vi "HFRR ADV v038 new software.vi"() -> ()   [LabVIEW 2025] (continued)
                            n2653 = local write "START TEMP"(w3137) -> ()
                            n2654 = local write "Remarks :"(w3139) -> ()
                            n2655 = local write "Main Dashboard Buttons"(T1."Imaging" ("Main Dashboard Buttons")) -> ()
                            n2656 = local write "Main Tab"(T2."Adv Scar" ("Main Tab")) -> ()
                            n2657 = property on="FRICVALZ 2" class="Bool (strict)"("DisabledEnum"=w3138) -> ()  [unwired: 2 in, 2 out]
                            n2658 = property on="FRICVALZ 3" class="Bool (strict)"("DisabledEnum"=w3138) -> ()  [unwired: 2 in, 2 out]
                            n2659 = property on="FRICVALZ 4" class="Bool (strict)"("DisabledEnum"=w3138) -> ()  [unwired: 2 in, 2 out]
                          }
                          frame #1 {
                            n2660 = Wait (ms)(milliseconds to wait=u32 1500) -> ()  [unwired: 1 out]
                          }
                          frame #2 {
                            n2661 = local read "WriteHumidity"() -> (w3153:string[])
                            n2662 = Insert Into Array(array=w3153, new element="R;1" ("new element/subarray")) -> (w3151:string[])  [unwired: 1 in]
                            n2663 = local write "Due Write"("VC;0") -> ()
                            n2664 = local write "WriteHumidity"(w3151) -> ()
                          }
                          frame #3 {
                            n2665 = Wait (ms)(milliseconds to wait=u32 1500) -> ()  [unwired: 1 out]
                          }
                          frame #4 {
                            n2666 = local read "WriteHumidity"() -> (w3158:string[])
                            n2667 = Insert Into Array(array=w3158, new element="R;1" ("new element/subarray")) -> (w3157:string[])  [unwired: 1 in]
                            n2668 = local write "Due Write"("VC;0") -> ()
                            n2669 = local write "WriteHumidity"(w3157) -> ()
                          }
                          frame #5 {
                            n2670 = Wait (ms)(milliseconds to wait=u32 1500) -> ()  [unwired: 1 out]
                          }
                          frame #6 {
                            n2671 = local write "Due Write"("ST;0") -> ()
                          }
                          frame #7 {
                            n2672 = local write "measured_stroke"(0.0 ("measured_stroke")) -> ()
                            n2673 = Wait (ms)(milliseconds to wait=u32 1500) -> ()  [unwired: 1 out]
                          }
                          frame #8 {
                            n2674 = local write "Humidity"(FALSE ("Humidity")) -> ()
                            n2675 = local write "Due Write"("HE;0") -> ()
                          }
                        }
                      }
                    }
                    n2676 = Divide(x=w3122, y=w3121) -> (x/y=w3125:dbl)
                    n2677 = Multiply(x=w3125, y=100.0) -> (x*y=w3123:dbl)
                    n2678 = local write "Test Duration Status"(w3123) -> ()
                  }
                }
              }
              frame #2 {
                n2679 = case shown="True" "Heater Button" {
                  tunnel: [0.0 ("output") w3265] -> w3243
                  frame False {
                    w3246 = TRUE ("tmpchk")
                    n2680 = local read "TEMP"() -> (w3247:dbl)
                    n2681 = local write "Temp ini"(w3247) -> ()
                    n2682 = local write "Reset 4"(w3246) -> ()
                    n2683 = local write "tmpchk"(w3246) -> ()
                    n2684 = local write "reinit"(TRUE ("reinit")) -> ()
                    n2685 = local write "manual temp log"(TRUE ("manual temp log")) -> ()
                  }
                  frame True {
                    # "Logic to turn off\nthe heater when \ntemp is not rising.\nTime - 60 sec\nDelta t- 5°c"
                    n2686 = local read "Temp ini"() -> (w3254:dbl)
                    n2687 = local read "Auto Start Test"() -> (w3250:bool)
                    n2688 = Less?(x=w3254, y=53.0) -> (x < y?=w3252:bool)
                    n2689 = case shown="False" w3250 {
                      frame False {
                        n2690 = local read "Set Temp"() -> (w3274:dbl)
                        n2691 = local read "TEMP"() -> (w3273:dbl)
                        n2692 = Subtract(x=w3274, y=w3273) -> (x-y=w3272:dbl)
                        n2693 = Absolute Value(x=w3272) -> (abs(x)=w3271:dbl)
                        n2694 = Less?(x=w3271, y=0.5) -> (x < y?=w3269:bool)
                        n2695 = case shown="True" w3269 {
                          tunnel: "manual temp log" -> [_ w3275]
                          frame False {
                          }
                          frame True {
                            n2696 = case shown="True" w3275 {
                              selector: w3275 -> [_ w3276]
                              frame False {
                              }
                              frame True {
                                # "#Event log"
                                n2697 = Not(x=w3276) -> (.not. x?=w3277:bool)
                                n2698 = local write "manual temp log"(w3277) -> ()
                                n2699 = local read "EVENT LOG"() -> (w3280:string)
                                n2700 = call "Event Log.vi"("Content"="Target Temperature reached", "EVENT LOG"=w3280) -> ("EVENT LOG"=w3279:string)  [unwired: 8 in, 1 out]
                                n2701 = local write "EVENT LOG"(w3279) -> ()
                              }
                            }
                          }
                        }
                      }
                      frame True {
                        n2702 = local write "manual temp log"(TRUE ("manual temp log")) -> ()
                      }
                    }
                    n2703 = And(x="tmpchk", y=w3252) -> (x .and. y?=w3255:bool)
                    n2704 = case shown="True" w3255 {
                      frame False {
                      }
                      frame True {
                        n2705 = call "Elapsed Time8"("Time Target (s)"=300.0, "Reset"="Reset 4") -> ("Time has Elapsed"=w3282:bool)  [unwired: 10 in, 7 out]
                        n2706 = flat-sequence {
                          tunnel: w3282 -> [_]
                          frame #0 {
                            n2707 = local write "Reset 4"(FALSE ("Reset 4")) -> ()
                          }
                        }
                        n2708 = case shown="True" w3282 {
                          frame False {
                          }
                          frame True {
                            n2709 = local read "Temp ini"() -> (w3289:dbl)
                            n2710 = Add(x=w3289, y=5.0) -> (x+y=w3287:dbl)
                            n2711 = local read "TEMP"() -> (w3290:dbl)
                            n2712 = Greater?(x=w3290, y=w3287) -> (0:w3288:bool)
                            n2713 = case shown="False" w3288 {
                              frame False {
                                n2714 = local write "Heater Button"(FALSE ("Heater Button")) -> ()
                              }
                              frame True {
                                n2715 = local write "tmpchk"(FALSE ("tmpchk")) -> ()
                              }
                            }
                          }
                        }
                      }
                    }
                    n2716 = local read "Set Temp"() -> (w3263:dbl)
                    n2717 = local read "TEMP"() -> (w3257:dbl)
                    n2718 = call-poly <vilib>:"PID.vi"("reinitialize? (F)"="reinit", "dt (s)"=-1.0, "process variable"=w3257, "setpoint"=w3263) -> ("output"=w3260:dbl)  [unwired: 6 in, 1 out]
                    n2719 = Subtract(x=w3263, y=w3257) -> (x-y=w3264:dbl)
                    n2720 = Add(x=w3263, y=0.5) -> (x+y=w3261:dbl)
                    n2721 = Greater Or Equal?(x=w3257, y=w3261) -> ()  [unwired: 1 out]
                    n2722 = Select(t=0.0, s=FALSE, f=w3260) -> (s? t:f=w3259:dbl)
                    "PID output" <- w3259
                    n2723 = flat-sequence {
                      tunnel: w3259 -> [w3293]
                      tunnel: [w3293] -> w3265
                      frame #0 {
                        n2724 = local write "reinit"(FALSE ("reinit")) -> ()
                      }
                    }
                    n2725 = Bundle(w3264, "output"=w3259, "TEMP"=w3257) -> ()  [unwired: 1 in, 1 out]
                  }
                }
                "PID-out" <- w3243
              }
              frame #3 {
                n2726 = local read "TEMP"() -> (w3295:dbl)
                n2727 = Greater Or Equal?(x=w3295, y="Set Temp 2") -> (x >= y?=w3300:bool)
                n2728 = case shown="True" w3300 {
                  tunnel: [FALSE TRUE] -> w3298
                  frame False {
                  }
                  frame True {
                  }
                }
                "Status 13" <- w3298
                n2729 = And(x=w3298, y="trip1 8") -> (x .and. y?=w3297:bool)
                n2730 = case shown="True" w3297 {
                  frame False {
                    n2731 = local write "Heater Trip Temp"(TRUE ("Heater Trip Temp")) -> ()
                  }
                  frame True {
                    w3303 = FALSE ("OK Button 2")
                    n2732 = case shown="True" "Heater Trip Temp" {
                      selector: "Heater Trip Temp" -> [_ w3305]
                      frame False {
                      }
                      frame True {
                        n2733 = Not(x=w3305) -> (.not. x?=w3304:bool)
                        n2734 = local read "EVENT LOG"() -> (w3308:string)
                        n2735 = local write "Heater Trip Temp"(w3304) -> ()
                        n2736 = call "Event Log.vi"("Content"="Heater Trip", "EVENT LOG"=w3308) -> ("EVENT LOG"=w3307:string)  [unwired: 8 in, 1 out]
                        n2737 = local write "EVENT LOG"(w3307) -> ()
                      }
                    }
                    n2738 = local write "RUN"(w3303) -> ()
                    n2739 = property on="Auto Start Test" class="Bool (strict)"("Value"=w3303) -> ()  [unwired: 2 in, 2 out]
                    n2740 = local write "Heater Button"(w3303) -> ()
                  }
                }
              }
            }
            n2741 = case shown="False" w3010 {
              frame False {
                n2742 = disable-structure shown="Disabled" {
                  frame Disabled {
                    n2743 = stacked-sequence {
                      frame #0 {
                        n2744 = local write "RUN"(FALSE ("OK Button 2")) -> ()
                      }
                      frame #1 {
                      }
                    }
                  }
                  frame Enabled {
                  }
                }
              }
              frame True {
              }
            }
          }
        }
        n2745 = local read "Reset Graph"() -> (w2903:bool)
        n2746 = case shown="True" w2903 {
          selector: w2903 -> [_ w2920]
          frame False {
          }
          frame True {
            w2934 = 0.0 ("X Scale.Range:Maximum")
            n2747 = Not(x=w2920) -> (.not. x?=w2919:bool)
            n2748 = local write "Reset Graph"(w2919) -> ()
            n2749 = property on="Electrical Contact Resistance ( % )" class="WFChart (strict)"("XScale.Maximum"=600.0 ("X Scale.Range:Maximum"), "XScale.Minimum"=0.0 ("X Scale.Range:Minimum"), "YScale.Maximum"=100.0 ("Y Scale.Range:Maximum"), "YScale.Minimum"=0.0 ("Y Scale.Range:Minimum")) -> ()  [unwired: 2 in, 2 out]
            n2750 = property on="Frictional Force ( N )" class="WFChart (strict)"("XScale.Maximum"=600.0 ("X Scale.Range:Maximum"), "XScale.Minimum"=0.0 ("X Scale.Range:Minimum"), "YScale.Maximum"=100.0 ("Y Scale.Range:Maximum"), "YScale.Minimum"=0.0 ("Y Scale.Range:Minimum")) -> ()  [unwired: 2 in, 2 out]
            n2751 = property on="Temperature ( Deg C )" class="WFChart (strict)"("XScale.Maximum"=600.0 ("X Scale.Range:Maximum"), "XScale.Minimum"=0.0 ("X Scale.Range:Minimum"), "YScale.Maximum"=100.0 ("Y Scale.Range:Maximum"), "YScale.Minimum"=0.0 ("Y Scale.Range:Minimum")) -> ()  [unwired: 2 in, 2 out]
            n2752 = property on="Stroke ( mm )" class="WFChart (strict)"("XScale.Maximum"=600.0 ("X Scale.Range:Maximum"), "XScale.Minimum"=0.0 ("X Scale.Range:Minimum"), "YScale.Maximum"=100.0 ("Y Scale.Range:Maximum"), "YScale.Minimum"=0.0 ("Y Scale.Range:Minimum")) -> ()  [unwired: 2 in, 2 out]
            n2753 = property on="Coefficient of Friction" class="WFChart (strict)"("XScale.Maximum"=600.0 ("X Scale.Range:Maximum"), "XScale.Minimum"=0.0 ("X Scale.Range:Minimum"), "YScale.Maximum"=100.0 ("Y Scale.Range:Maximum"), "YScale.Minimum"=0.0 ("Y Scale.Range:Minimum")) -> ()  [unwired: 2 in, 2 out]
            n2754 = property on="Electrical Contact Resistance ( % )" class="WFChart (strict)"("XScale.Minimum"=0.0 ("X Scale.Range:Minimum"), "XScale.Maximum"=600.0 ("X Scale.Range:Maximum"), "YScale.Minimum"=0.0 ("Y Scale.Range:Minimum"), "YScale.Maximum"=100.0 ("Y Scale.Range:Maximum")) -> ()  [unwired: 2 in, 2 out]
            n2755 = property on="Temperature ( Deg C )" class="WFChart (strict)"("XScale.Minimum"=0.0 ("X Scale.Range:Minimum"), "XScale.Maximum"=600.0 ("X Scale.Range:Maximum"), "YScale.Minimum"=0.0 ("Y Scale.Range:Minimum"), "YScale.Maximum"=100.0 ("Y Scale.Range:Maximum")) -> ()  [unwired: 2 in, 2 out]
            n2756 = property on="Coefficient of Friction" class="WFChart (strict)"("XScale.Minimum"=0.0 ("X Scale.Range:Minimum"), "XScale.Maximum"=600.0 ("X Scale.Range:Maximum"), "YScale.Maximum"=1.0 ("X Scale.Range:Minimum"), "YScale.Minimum"=0.0 ("X Scale.Range:Minimum")) -> ()  [unwired: 2 in, 2 out]
            n2757 = property on="Frictional Force ( N )" class="WFChart (strict)"("XScale.Maximum"=600.0 ("X Scale.Range:Maximum"), "XScale.Minimum"=w2934, "YScale.Maximum"=10.0 ("Y Scale.Range:Maximum"), "YScale.Minimum"=w2934) -> ()  [unwired: 2 in, 2 out]
            n2758 = property on="Stroke ( mm )" class="WFChart (strict)"("XScale.Maximum"=600.0 ("X Scale.Range:Maximum"), "XScale.Minimum"=0.0 ("X Scale.Range:Minimum"), "YScale.Maximum"=100.0 ("Y Scale.Range:Maximum"), "YScale.Minimum"=0.0 ("Y Scale.Range:Minimum")) -> ()  [unwired: 2 in, 2 out]
            n2759 = property on="Humidity ( %RH ) 2" class="WFChart (strict)"("XScale.Maximum"=600.0 ("X Scale.Range:Maximum"), "XScale.Minimum"=0.0 ("X Scale.Range:Minimum"), "YScale.Maximum"=100.0 ("Y Scale.Range:Maximum"), "YScale.Minimum"=0.0 ("Y Scale.Range:Minimum")) -> ()  [unwired: 2 in, 2 out]
          }
        }
      }
      frame "Compare Files" {
        # "Elapsed time\ncof\nstroke\nAir temp\nTemp\nHumidity"
        n2760 = case shown="True" "RSTV1 2" {
          frame False {
          }
          frame True {
            n2761 = property on="Humidity ( %RH )" class="XYGraph (strict)"("Y Scale.Display Format:Precision"=u8 0 ("Y Scale.Format & Precision:Precision")) -> ()  [unwired: 2 in, 2 out]
            n2762 = property on="Humidity ( %RH )" class="XYGraph (strict)"("X Scale.Range:Minimum"=0.0, "X Scale.Range:Maximum"=75.0, "Y Scale.Range:Minimum"=48.0, "Y Scale.Range:Maximum"=58.0) -> ()  [unwired: 2 in, 2 out]
          }
        }
        n2763 = case shown="True" "RST CP 2" {
          frame False {
          }
          frame True {
            n2764 = property on="XY Graph 13" class="XYGraph (strict)"("Y Scale.Display Format:Precision"=u8 0 ("Y Scale.Format & Precision:Precision")) -> ()  [unwired: 2 in, 2 out]
            n2765 = property on="XY Graph 13" class="XYGraph (strict)"("X Scale.Range:Minimum"=0.0, "X Scale.Range:Maximum"=75.0, "Y Scale.Range:Minimum"=0.0, "Y Scale.Range:Maximum"=100.0) -> ()  [unwired: 2 in, 2 out]
          }
        }
        n2766 = case shown="True" "RST CP" {
          frame False {
          }
          frame True {
            n2767 = property on="Sample Temperature ( °C )" class="XYGraph (strict)"("Y Scale.Display Format:Precision"=u8 2 ("Y Scale.Format & Precision:Precision")) -> ()  [unwired: 2 in, 2 out]
            n2768 = property on="Sample Temperature ( °C )" class="XYGraph (strict)"("X Scale.Range:Minimum"=0.0, "X Scale.Range:Maximum"=75.0, "Y Scale.Range:Minimum"=58.0, "Y Scale.Range:Maximum"=62.0) -> ()  [unwired: 2 in, 2 out]
          }
        }
        n2769 = case shown="True" "RSTV1 3" {
          frame False {
          }
          frame True {
            n2770 = property on="Air Temperature  ( °C )" class="XYGraph (strict)"("Y Scale.Display Format:Precision"=u8 2 ("Y Scale.Format & Precision:Precision")) -> ()  [unwired: 2 in, 2 out]
            n2771 = property on="Air Temperature  ( °C )" class="XYGraph (strict)"("X Scale.Range:Minimum"=0.0 ("Y Scale.Range:Minimum"), "X Scale.Range:Maximum"=75.0 ("Y Scale.Range:Maximum"), "Y Scale.Range:Minimum"=20.0 ("X Scale.Range:Minimum"), "Y Scale.Range:Maximum"=26.0 ("X Scale.Range:Maximum")) -> ()  [unwired: 2 in, 2 out]
          }
        }
        n2772 = case shown="True" "RSTV1 4" {
          frame False {
          }
          frame True {
            n2773 = property on="Stroke ( mm )" class="XYGraph (strict)"("Y Scale.Display Format:Precision"=u8 2 ("Y Scale.Format & Precision:Precision")) -> ()  [unwired: 2 in, 2 out]
            n2774 = property on="Stroke ( mm )" class="XYGraph (strict)"("X Scale.Range:Minimum"=0.0 ("Y Scale.Range:Maximum"), "X Scale.Range:Maximum"=75.0 ("X Scale.Range:Minimum"), "Y Scale.Range:Minimum"=0.98, "Y Scale.Range:Maximum"=1.02) -> ()  [unwired: 2 in, 2 out]
          }
        }
        n2775 = case shown="True" "rstv2" {
          frame False {
          }
          frame True {
            n2776 = property on="Coefficient Of Friction" class="XYGraph (strict)"("Y Scale.Display Format:Precision"=u8 3 ("Y Scale.Format & Precision:Precision")) -> ()  [unwired: 2 in, 2 out]
            n2777 = property on="Coefficient Of Friction" class="XYGraph (strict)"("X Scale.Range:Minimum"=0.0 ("Y Scale.Range:Maximum"), "X Scale.Range:Maximum"=75.0, "Y Scale.Range:Minimum"=0.0, "Y Scale.Range:Maximum"=1.0 ("X Scale.Range:Minimum")) -> ()  [unwired: 2 in, 2 out]
          }
        }
        n2778 = case shown="True" "RST CP 3" {
          frame False {
          }
          frame True {
            n2779 = property on="Air Temp ( °C ) vs Humidity ( % RH )" class="XYGraph (strict)"("X Scale.Range:Minimum"=18.0, "X Scale.Range:Maximum"=28.0 ("X Scale.Range:Minimum"), "Y Scale.Range:Minimum"=30.0 ("X Scale.Range:Minimum"), "Y Scale.Range:Maximum"=70.0 ("X Scale.Range:Minimum")) -> ()  [unwired: 2 in, 2 out]
          }
        }
        n2780 = case shown="True" "OPEN 1" {
          frame False {
          }
          frame True {
            (unwired) 0  # existing file
            w3584 = "Choose a datalog file to open"  # prompt
            n2781 = local write "OPEN 1"(FALSE ("OPEN 1")) -> ()
            n2782 = String To Path(string="C:\\LAB-IQ\\Data\\") -> (path=w3569:path)
            n2783 = File Dialog(6:"*.dgf" ("pattern"), 7:w3584, 11:w3569) -> (0:w3567:errorcluster, 3:w3575:path)  [unwired: 4 in, 2 out]
            n2784 = Unbundle(w3567) -> ()  [unwired: 3 out]
            n2785 = Strip Path(path=w3575) -> (name=w3574:string)  [unwired: 1 out]
            n2786 = Path To String(path=w3575) -> (string=w3570:string)
            "string1" <- w3570
            n2787 = Match Pattern(string=w3574, regular expression=".dgf") -> (before substring=→"String Control":string)  [unwired: 1 in, 3 out]
            n2788 = Match Pattern(string=w3570, regular expression=".dgf" ("substring (\"\")")) -> (before substring=w3580:string)  [unwired: 1 in, 3 out]
            n2789 = Concatenate Strings(w3580, ".duf" ("Substring")) -> (w3576:string)
            n2790 = String To Path(string=w3576) -> (path=w3581:path)
            n2791 = call <vilib>:"Read Characters From File.vi"("file path (dialog if empty)"=w3581, "start of read offset (chars.:0)"=60 ("start of read offset (chars.: 0)")) -> ("character string"=→"String Control 2":string)  [unwired: 4 in, 3 out]
          }
        }
        n2792 = case shown="True" "OPEN 2" {
          frame False {
          }
          frame True {
            (unwired) 0  # existing file
            w3602 = "Choose a datalog file to open"  # prompt
            n2793 = local write "OPEN 2"(FALSE ("OPEN 1")) -> ()
            n2794 = String To Path(string="C:\\LAB-IQ\\Data\\") -> (path=w3587:path)
            n2795 = File Dialog(6:"*.dgf" ("pattern"), 7:w3602, 11:w3587) -> (0:w3585:errorcluster, 3:w3593:path)  [unwired: 4 in, 2 out]
            n2796 = Unbundle(w3585) -> ()  [unwired: 3 out]
            n2797 = Strip Path(path=w3593) -> (name=w3591:string)  [unwired: 1 out]
            n2798 = Path To String(path=w3593) -> (string=w3588:string)
            "string1 2" <- w3588
            n2799 = Match Pattern(string=w3591, regular expression=".dgf") -> (before substring=→"String Control 3":string)  [unwired: 1 in, 3 out]
            n2800 = Match Pattern(string=w3588, regular expression=".dgf" ("substring (\"\")")) -> (before substring=w3599:string)  [unwired: 1 in, 3 out]
            n2801 = Concatenate Strings(w3599, ".duf" ("Substring")) -> (w3596:string)
            n2802 = String To Path(string=w3596) -> (path=w3594:path)
            n2803 = call <vilib>:"Read Characters From File.vi"("file path (dialog if empty)"=w3594, "start of read offset (chars.:0)"=60 ("start of read offset (chars.: 0)")) -> ("character string"=→"String Control 4":string)  [unwired: 4 in, 3 out]
          }
        }
        n2804 = case shown="True" "OPEN 3" {
          frame False {
          }
          frame True {
            (unwired) 0  # existing file
            w3620 = "Choose a datalog file to open"  # prompt
            n2805 = local write "OPEN 3"(FALSE ("OPEN 1")) -> ()
            n2806 = String To Path(string="C:\\LAB-IQ\\Data\\") -> (path=w3605:path)
            n2807 = File Dialog(6:"*.dgf" ("pattern"), 7:w3620, 11:w3605) -> (0:w3603:errorcluster, 3:w3611:path)  [unwired: 4 in, 2 out]
            n2808 = Unbundle(w3603) -> ()  [unwired: 3 out]
            n2809 = Strip Path(path=w3611) -> (name=w3609:string)  [unwired: 1 out]
            n2810 = Path To String(path=w3611) -> (string=w3606:string)
            "string1 3" <- w3606
            n2811 = Match Pattern(string=w3609, regular expression=".dgf") -> (before substring=→"String Control 5":string)  [unwired: 1 in, 3 out]
            n2812 = Match Pattern(string=w3606, regular expression=".dgf" ("substring (\"\")")) -> (before substring=w3616:string)  [unwired: 1 in, 3 out]
            n2813 = Concatenate Strings(w3616, ".duf" ("Substring")) -> (w3613:string)
            n2814 = String To Path(string=w3613) -> (path=w3617:path)
            n2815 = call <vilib>:"Read Characters From File.vi"("file path (dialog if empty)"=w3617, "start of read offset (chars.:0)"=60 ("start of read offset (chars.: 0)")) -> ("character string"=→"String Control 6":string)  [unwired: 4 in, 3 out]
          }
        }
        n2816 = case shown="True" "OPEN 4" {
          frame False {
          }
          frame True {
            (unwired) 0  # existing file
            w3638 = "Choose a datalog file to open"  # prompt
            n2817 = local write "OPEN 4"(FALSE ("OPEN 1")) -> ()
            n2818 = String To Path(string="C:\\LAB-IQ\\Data\\") -> (path=w3623:path)
            n2819 = File Dialog(6:"*.dgf" ("pattern"), 7:w3638, 11:w3623) -> (0:w3621:errorcluster, 3:w3629:path)  [unwired: 4 in, 2 out]
            n2820 = Unbundle(w3621) -> ()  [unwired: 3 out]
            n2821 = Strip Path(path=w3629) -> (name=w3627:string)  [unwired: 1 out]
            n2822 = Path To String(path=w3629) -> (string=w3624:string)
            "string1 4" <- w3624
            n2823 = Match Pattern(string=w3627, regular expression=".dgf") -> (before substring=→"String Control 7":string)  [unwired: 1 in, 3 out]
            n2824 = Match Pattern(string=w3624, regular expression=".dgf" ("substring (\"\")")) -> (before substring=w3634:string)  [unwired: 1 in, 3 out]
            n2825 = Concatenate Strings(w3634, ".duf" ("Substring")) -> (w3631:string)
            n2826 = String To Path(string=w3631) -> (path=w3635:path)
            n2827 = call <vilib>:"Read Characters From File.vi"("file path (dialog if empty)"=w3635, "start of read offset (chars.:0)"=60 ("start of read offset (chars.: 0)")) -> ("character string"=→"String Control 8":string)  [unwired: 4 in, 3 out]
          }
        }
      }
      frame "About" {
        # "Elapsed time\ncof\nstroke\nmean pos\nTemp\nHumidity"
        n2828 = disable-structure shown="Disabled" {
          frame Disabled {
            n2829 = case shown="True" "Export" {
              frame False {
              }
              frame True {
                w3660 = "                                      " ("string")
                w3662 = "\r"
                (unwired) i16 6 ("width (-)")
                w3739 = "\r"
                w3671 = "\r"
                n2830 = local write "Export"(FALSE ("Export")) -> ()
                n2831 = local read "String 29"() -> (w3708:string)
                n2832 = local read "String 34"() -> (w3696:string)
                n2833 = local read "String 35"() -> (w3691:string)
                n2834 = local read "String 37"() -> (w3687:string)
                n2835 = local read "String 36"() -> (w3684:string)
                n2836 = local read "String 38"() -> (w3681:string)
                n2837 = local read "String 39"() -> (w3678:string)
                n2838 = Match Pattern(string=w3708, regular expression=".dwm") -> (before substring=w3704:string)  [unwired: 1 in, 3 out]
                "before substring" <- w3704
                n2839 = local read "S 38"() -> (w3699:string)
                n2840 = local read "S 39"() -> (w3692:string)
                n2841 = local read "Temperature before test 2"() -> (w3728:dbl)
                n2842 = local read "Temperature after test 2"() -> (w3733:dbl)
                n2843 = local read "Humidity before test 2"() -> (w3714:dbl)
                n2844 = local read "Humidity after test 2"() -> (w3729:dbl)
                n2845 = local read "MWSD 2"() -> (w3725:dbl)
                n2846 = local read "WS1.4 2"() -> (w3741:dbl)
                n2847 = local read "HCF 2"() -> (w3737:dbl)
                n2848 = local read "AVP 2"() -> (w3726:dbl)
                n2849 = Concatenate Strings("1," ("string"), w3699) -> (w3698:string)
                n2850 = Concatenate Strings("2," ("string"), w3696) -> (w3695:string)
                n2851 = Concatenate Strings("3," ("string"), w3692) -> (w3694:string)
                n2852 = Concatenate Strings("4," ("string"), w3691) -> (w3690:string)
                n2853 = Concatenate Strings("5," ("string"), w3687) -> (w3688:string)
                n2854 = Concatenate Strings("6," ("string"), w3684) -> (w3685:string)
                n2855 = Concatenate Strings("7," ("string"), w3681) -> (w3682:string)
                n2856 = Concatenate Strings("8," ("string"), w3678) -> (w3679:string)
                n2857 = local read "Sample ID"() -> (w3746:string)
                n2858 = case shown="\"xlx\"" "Select File Type" {
                  tunnel: w3704 -> [w3749 w3751 w3753]
                  tunnel: [w3747 w3752 w3754] -> w3703
                  frame "xlx" {
                    n2859 = Concatenate Strings(w3749, ".xls" ("string")) -> (w3747:string)
                  }
                  frame "csv" {
                    n2860 = Concatenate Strings(w3751, ".csv" ("string")) -> (w3752:string)
                  }
                  frame "txt" {
                    n2861 = Concatenate Strings(w3753, ".txt" ("string")) -> (w3754:string)
                  }
                }
                n2862 = local read "Test Date"() -> (w3745:string)
                n2863 = local read "String 45"() -> (w3659:string)
                n2864 = local read "String 31"() -> (w3744:string)
                n2865 = local read "String 32"() -> (w3743:string)
                n2866 = local read "TITTLE"() -> (w3667:string)
                n2867 = Number To Fractional String(number=w3714, width (-)=i16 6, precision (6)=i16 2) -> (F-format string=w3713:string)  [unwired: 1 in]
                n2868 = Number To Fractional String(number=w3728, width (-)=i16 6, precision (6)=i16 2) -> (F-format string=w3734:string)  [unwired: 1 in]
                n2869 = Number To Fractional String(number=w3729, width (-)=i16 6, precision (6)=i16 2) -> (F-format string=w3727:string)  [unwired: 1 in]
                n2870 = Number To Fractional String(number=w3733, width (-)=i16 6, precision (6)=i16 2) -> (F-format string=w3732:string)  [unwired: 1 in]
                n2871 = Number To Fractional String(number=w3725, width (-)=i16 6, precision (6)=i16 2) -> (F-format string=w3723:string)  [unwired: 1 in]
                n2872 = Number To Fractional String(number=w3726, width (-)=i16 6, precision (6)=i16 2) -> (F-format string=w3724:string)  [unwired: 1 in]
                n2873 = Number To Fractional String(number=w3737, width (-)=i16 6, precision (6)=i16 2) -> (F-format string=w3738:string)  [unwired: 1 in]
                n2874 = Number To Fractional String(number=w3741, precision (6)=i16 2) -> (F-format string=w3742:string)  [unwired: 2 in]
                n2875 = local read "s.NO"() -> (w3661:string)
                n2876 = Concatenate Strings("=" ("string"), w3667) -> (w3666:string)
                n2877 = Concatenate Strings("S.No," ("string"), "                                       Parameters" ("string")) -> (w3672:string)
                n2878 = Concatenate Strings(w3739, w3698, w3713, w3739, w3695, w3734, w3739, w3694, w3727, w3739, w3690, w3732, w3739, w3688, w3723, w3739, w3685, w3724, w3739, w3682, w3738, w3739, w3679, w3742) -> (w3701:string)
                n2879 = Concatenate Strings(w3671, "," ("string"), w3659, w3661, w3660, w3743, w3746, w3660, w3744, w3745, w3671) -> (w3669:string)
                n2880 = local read "Tested by"() -> (w3675:string)
                n2881 = local read "String 33"() -> (w3676:string)
                n2882 = Concatenate Strings("," ("string"), "                                                                             " ("string")) -> (w3664:string)
                n2883 = Concatenate Strings(w3666, w3662, w3669, w3662, w3672, w3701, w3662, w3664, w3676, w3675) -> (→"export":string)
                n2884 = String To Path(string=w3703) -> (path=w3710:path)
                n2885 = local read "export"() -> (w3705:string)
                n2886 = call <vilib>:"Write Characters To File.vi"("append to file? (new file:F)"=FALSE, "character string"=w3705, "file path (dialog if empty)"=w3710) -> ()  [unwired: 2 in, 1 out]
              }
            }
          }
          frame Enabled {
          }
        }
        n2887 = case shown="True" "OK Button 17" {
          frame False {
          }
          frame True {
            (unwired) 0  # existing file
            w3963 = "Choose a datalog file to open"  # prompt
            n2888 = local write "OK Button 17"(FALSE ("OK Button 17")) -> ()
            n2889 = local read "String"() -> (w3958:string)
            n2890 = String To Path(string=w3958) -> (path=w3959:path)
            n2891 = File Dialog(6:"*.duf" ("pattern"), 7:w3963, 11:w3959) -> (0:w3950:errorcluster, 3:w3969:path)  [unwired: 4 in, 2 out]
            n2892 = Unbundle(w3950) -> ()  [unwired: 3 out]
            n2893 = Open/Create/Replace File "Open File"(file path (use dialog)=w3969) -> (refnum out=w3961:refnum<file>)  [unwired: 5 in, 2 out]
            n2894 = Strip Path(path=w3969) -> (name=w3967:string)  [unwired: 1 out]
            n2895 = Path To String(path=w3969) -> (string=w3952:string)
            n2896 = while {
              tunnel: w3961 -> [w3973]
              i -> [w3970]
              stop <- w3971 continue-if-true
              (unwired) TRUE ("line mode (F)")
              n2897 = Read from Text File "Read File"(file (use dialog)=w3973) -> (text=w3972:string)  [unwired: 3 in, 3 out]
              n2898 = local write "Numeric 16"(w3970) -> ()
              n2899 = String Length(string=w3972) -> (length=w3975:i32)
              n2900 = Greater?(x=w3975, y=1) -> (0:w3971:bool)
            }
            n2901 = local write "String 29"(w3952) -> ()
            n2902 = Search and Replace String(input string=w3952, search string=".duf", replace string=".dgf" ("replace string (\"\")")) -> (result string=→"String Indicator 4":string)  [unwired: 5 in, 3 out]
            n2903 = Match Pattern(string=w3967, regular expression=".dwm") -> (before substring=w3951:string)  [unwired: 1 in, 3 out]
            "String Indicator" <- w3951
            n2904 = Match Pattern(string=w3952, regular expression=".dwm" ("substring (\"\")")) -> (before substring=w3953:string)  [unwired: 1 in, 3 out]
            "String Indicator 3" <- w3953
            n2905 = local write "TITTLE 2"(w3951) -> ()
            n2906 = String To Path(string=w3953) -> (path=w3960:path)
            "path" <- w3960
            n2907 = call <vilib>:"Read Characters From File.vi"("file path (dialog if empty)"=w3960, "start of read offset (chars.:0)"=60 ("start of read offset (chars.: 0)")) -> ("character string"=→"String Indicator 2":string)  [unwired: 4 in, 3 out]
          }
        }
        n2908 = call <vilib>:"Query Available Printers.vi"() -> ("system configured printers"=w3652:string[])  [unwired: 9 in, 2 out]
        "System Configured Printers 2" <- w3652
        n2909 = local read "OK Button 16"() -> (w3649:bool)
        n2910 = case shown="True" "OK Button 16" {
          frame False {
          }
          frame True {
            n2911 = stacked-sequence {
              frame #0 {
                n2912 = local read "Numeric 16"() -> (w3977:i32)
                n2913 = local write "Numeric 10"(w3977) -> ()
              }
              frame #1 {
                n2914 = local read "String 29"() -> (w3980:string)
                n2915 = String To Path(string=w3980) -> (path=w3979:path)
                n2916 = Open/Create/Replace File "Open File"(file path (use dialog)=w3979) -> (refnum out=w3981:refnum<file>)  [unwired: 5 in, 2 out]
                n2917 = for {
                  N: 16 -> [_]
                  tunnel: w3981 -> [w3988]
                  i -> [w3984]
                  (unwired) TRUE ("line mode (F)")
                  n2918 = Read from Text File "Read File"(file (use dialog)=w3988) -> (text=w3982:string)  [unwired: 3 in, 3 out]
                  n2919 = Match Pattern(string=w3982, regular expression="(") -> (after substring=w3987:string)  [unwired: 1 in, 3 out]
                  n2920 = Match Pattern(string=w3987, regular expression=")") -> (before substring=w3983:string)  [unwired: 1 in, 3 out]
                  n2921 = case shown="1" w3984 {
                    tunnel: w3983 -> [w3989 w3990 _ _ w3991 w3992 w3993 w3995 w3997 w3999 w4001 w4003 w4005 w4007 _]
                    tunnel: w3982 -> [_ _ _ _ _ _ _ _ _ _ _ _ _ _ _]
                    frame 0 {
                      "TITTLE" <- w3989
                    }
                    frame 1 {
                      "Sample ID" <- w3990
                    }
                    frame 2 {
                    }
                    frame 3 {
                    }
                    frame 4 {
                      "Test Date" <- w3991
                    }
                    frame 5 {
                      "Tested by" <- w3992
                    }
                    frame 6 {
                      n2922 = Fract/Exp String To Number(string=w3993) -> (number=→"Humidity before test 2":dbl)  [unwired: 3 in, 1 out]
                    }
                    frame 7 {
                      n2923 = Fract/Exp String To Number(string=w3995) -> (number=→"Temperature before test 2":dbl)  [unwired: 3 in, 1 out]
                    }
                    frame 8 {
                      n2924 = Fract/Exp String To Number(string=w3997) -> (number=→"Humidity after test 2":dbl)  [unwired: 3 in, 1 out]
                    }
                    frame 9 {
                      n2925 = Fract/Exp String To Number(string=w3999) -> (number=→"Temperature after test 2":dbl)  [unwired: 3 in, 1 out]
                    }
                    frame 10 {
                      n2926 = Fract/Exp String To Number(string=w4001) -> (number=→"MWSD 2":dbl)  [unwired: 3 in, 1 out]
                    }
                    frame 11 {
                      n2927 = Fract/Exp String To Number(string=w4003) -> (number=→"AVP 2":dbl)  [unwired: 3 in, 1 out]
                    }
                    frame 12 {
                      n2928 = Fract/Exp String To Number(string=w4005) -> (number=→"HCF 2":dbl)  [unwired: 3 in, 1 out]
                    }
                    frame 13 {
                      n2929 = Fract/Exp String To Number(string=w4007) -> (number=→"WS1.4 2":dbl)  [unwired: 3 in, 1 out]
                    }
                    frame 14, Default {
                    }
                  }
                }
              }
              frame #2 {
              }
            }
            n2930 = local write "OK Button 16"(FALSE ("OK Button 13")) -> ()
          }
        }
        n2931 = Index Array(array=w3652, index="Select Printer 3") -> (element=w3654:string)
        "Selected Printer" <- w3654
        n2932 = case shown="True" w3649 {
          frame False {
          }
          frame True {
            n2933 = flat-sequence {
              frame #0 {
              }
              frame #1 {
                n2934 = Wait (ms)(milliseconds to wait=u32 100) -> ()  [unwired: 1 out]
              }
              frame #2 {
                n2935 = local write "OK Button 16"(FALSE ("Print 3")) -> ()
              }
            }
          }
        }
        n2936 = case shown="True" "Print" {
          tunnel: w3654 -> [_ w3946]
          frame False {
          }
          frame True {
            (unwired) i16 6 ("width (-)")
            (unwired) "TESTED BY : "
            (unwired) "TESTED DATE :"
            (unwired) "SAMPLE ID : "
            (unwired) "SAMPLE DESIGN : "
            w3904 = "\r"
            w3921 = "\r"
            # "add image"
            n2937 = local read "Sample ID"() -> (w3894:string)
            n2938 = local read "Tested by"() -> (w3897:string)
            n2939 = local read "String 34"() -> (w3884:string)
            n2940 = local read "String 45"() -> (w3864:string)
            n2941 = local read "String 35"() -> (w3879:string)
            n2942 = local read "String 37"() -> (w3877:string)
            n2943 = local read "String 32"() -> (w3899:string)
            n2944 = local read "String 36"() -> (w3874:string)
            n2945 = local read "String 31"() -> (w3898:string)
            n2946 = local read "Test Date"() -> (w3895:string)
            n2947 = local read "String 33"() -> (w3900:string)
            n2948 = local read "String 38"() -> (w3870:string)
            n2949 = local read "String 39"() -> (w3867:string)
            n2950 = local write "Print"(FALSE ("Print FF")) -> ()
            n2951 = local read "S 39"() -> (w3882:string)
            n2952 = local read "S 38"() -> (w3889:string)
            n2953 = local read "Temperature before test 2"() -> (w3920:dbl)
            n2954 = local read "Temperature after test 2"() -> (w3910:dbl)
            n2955 = local read "Humidity before test 2"() -> (w3935:dbl)
            n2956 = local read "Humidity after test 2"() -> (w3919:dbl)
            n2957 = local read "MWSD 2"() -> (w3924:dbl)
            n2958 = local read "WS1.4 2"() -> (w3902:dbl)
            n2959 = Concatenate Strings("2)" ("string"), w3884) -> (w3885:string)
            n2960 = Concatenate Strings("3)" ("string"), w3882) -> (w3883:string)
            n2961 = Concatenate Strings("1)" ("string"), w3889) -> (w3888:string)
            n2962 = Concatenate Strings("4)" ("string"), w3879) -> (w3880:string)
            n2963 = Concatenate Strings("5)" ("string"), w3877) -> (w3876:string)
            n2964 = Concatenate Strings("6)" ("string"), w3874) -> (w3873:string)
            n2965 = Concatenate Strings("7)" ("string"), w3870) -> (w3871:string)
            n2966 = Concatenate Strings("8)" ("string"), w3867) -> (w3868:string)
            n2967 = local read "HCF 2"() -> (w3906:dbl)
            n2968 = local read "AVP 2"() -> (w3923:dbl)
            n2969 = local read "s.NO"() -> (w3865:string)
            n2970 = call <vilib>:"New Report.vi"("report type"=enum16{"Standard Report", "HTML"}."Standard Report") -> ("report out"=w3944:refnum<class "NI_report.lvclass">, "error out"=w3943:errorcluster)  [unwired: 13 in]
            n2971 = local read "TITTLE"() -> (w3896:string)
            n2972 = Concatenate Strings(w3921, w3864, w3865, w3921, w3899, w3894, w3921, w3898, w3895, w3921, w3900, w3897, w3921) -> (w3914:string)
            "test by" <- w3914
            n2973 = Number To Fractional String(number=w3920, width (-)=i16 6, precision (6)=i16 2) -> (F-format string=w3909:string)  [unwired: 1 in]
            n2974 = Number To Fractional String(number=w3919, width (-)=i16 6, precision (6)=i16 2) -> (F-format string=w3922:string)  [unwired: 1 in]
            n2975 = Number To Fractional String(number=w3935, width (-)=i16 6, precision (6)=i16 2) -> (F-format string=w3940:string)  [unwired: 1 in]
            n2976 = Number To Fractional String(number=w3924, width (-)=i16 6, precision (6)=i16 2) -> (F-format string=w3926:string)  [unwired: 1 in]
            n2977 = Number To Fractional String(number=w3910, width (-)=i16 6, precision (6)=i16 2) -> (F-format string=w3911:string)  [unwired: 1 in]
            n2978 = Number To Fractional String(number=w3923, width (-)=i16 6, precision (6)=i16 2) -> (F-format string=w3925:string)  [unwired: 1 in]
            n2979 = Number To Fractional String(number=w3906, width (-)=i16 6, precision (6)=i16 2) -> (F-format string=w3905:string)  [unwired: 1 in]
            n2980 = Number To Fractional String(number=w3902, precision (6)=i16 2) -> (F-format string=w3901:string)  [unwired: 2 in]
            n2981 = call-dynamic "Set Report Header Text.vi"("report in"=w3944, "center header text"=w3896, "error in (no error)"=w3943) -> ("report out"=w3915:refnum<class "NI_report.lvclass">, "error out"=w3916:errorcluster)  [unwired: 11 in]
            n2982 = Concatenate Strings(w3904, w3888, w3940, w3904, w3885, w3909, w3904, w3883, w3922, w3904, w3880, w3911, w3904, w3876, w3926, w3904, w3873, w3925, w3904, w3871, w3905, w3904, w3868, w3901) -> (w3892:string)
            "export 2" <- w3892
            n2983 = call-poly <vilib>:"Append Report Text.vi"("report in"=w3915, "text"=w3914, "error in (no error)"=w3916) -> ("report out"=w3918:refnum<class "NI_report.lvclass">, "error out"=w3917:errorcluster)  [unwired: 9 in, 2 out]
            n2984 = local read "test by"() -> (w3891:string)
            n2985 = local read "TITTLE"() -> (w3893:string)
            n2986 = call-poly <vilib>:"Append Report Text.vi"("report in"=w3918, "error in (no error)"=w3917) -> ("report out"=w3939:refnum<class "NI_report.lvclass">, "error out"=w3937:errorcluster)  [unwired: 10 in, 2 out]
            n2987 = Concatenate Strings(w3893, w3892, w3891) -> (→"output":string)
            n2988 = call-poly <vilib>:"Append Report Text.vi"("report in"=w3939, "text"=w3892, "error in (no error)"=w3937) -> ("report out"=w3938:refnum<class "NI_report.lvclass">, "error out"=w3936:errorcluster)  [unwired: 9 in, 2 out]
            n2989 = call-dynamic "Print Report.vi"("report in"=w3938, "printer name (default)"=w3946, "error in (no error)"=w3936) -> ("report out"=w3948:refnum<class "NI_report.lvclass">, "error out"=w3949:errorcluster)  [unwired: 11 in]
            n2990 = call-dynamic "Dispose Report.vi"("report in"=w3948, "error in (no error)"=w3949) -> ()  [unwired: 13 in, 1 out]
          }
        }
        n2991 = case shown="True" "Print 2" {
          frame False {
          }
          frame True {
            n2992 = flat-sequence {
              frame #0 {
                n2993 = local read "s.NO"() -> (→"s.NO 2":string)
                n2994 = Wait (ms)(milliseconds to wait=u32 20) -> ()  [unwired: 1 out]
                n2995 = local read "Sample ID  3"() -> (→"Sample ID  6":string)
                n2996 = local read "Sample ID  4"() -> (→"Sample ID  7":string)
                n2997 = local read "Sample ID"() -> (→"Sample ID  2":string)
                n2998 = local read "Tested by"() -> (→"Tested by 2":string)
                n2999 = local read "Test Date"() -> (→"Test Date 2":string)
                n3000 = local read "Humidity after test 3"() -> (→"Humidity after test 4":dbl)
                n3001 = local read "Ref A Test Date :"() -> (→"TITTLE 4":string)
                n3002 = local read "Temperature before test 3"() -> (w3771:dbl)
                n3003 = local read "Temperature before test 3"() -> (→"Temperature after test 5":dbl)
                n3004 = local read "Temperature after test 3"() -> (→"Temperature after test 4":dbl)
                n3005 = local read "Humidity before test 3"() -> (→"Humidity before test 4":dbl)
                n3006 = local write "Temperature before test 3"(w3771) -> ()
                n3007 = local read "image data"() -> (w3762:T16)
                n3008 = String To Path(string="C:\\LAB-IQ\\im\\Temp_resized.jpg") -> (path=w3763:path)
                "path 2" <- w3763
                n3009 = call <vilib>:"Write JPEG File.vi"("image data"=w3762, "path to JPEG file"=w3763) -> ()  [unwired: 8 in, 2 out]
                "Ref A Test Date :" <- "Ref A Test Date :"
                "Ref B Test Date :" <- "Ref B Test Date :"
                "Ref B Scar Value :" <- "Ref B Scar Value :"
                "Ref A Scar Value :" <- "Ref A Scar Value :"
              }
              frame #1 {
                (unwired) HTML_Report_Image_Alignment."MIDDLE" ("alignment (default)")
                w3799 = u16 0 items=["portrait", "landscape"] ("orientation (portrait)")
                (unwired) HTML_Report_Image_Alignment."ABSMIDDLE" ("alignment (default)")
                (unwired) "TESTED BY : "
                (unwired) "TESTED DATE :"
                (unwired) "SAMPLE ID : "
                (unwired) "SAMPLE DESIGN : "
                w3832 = "\r"
                # "add image"
                n3010 = Wait (ms)(milliseconds to wait=u32 20) -> ()  [unwired: 1 out]
                n3011 = local read "Sample ID  2"() -> (w3825:string)
                n3012 = local read "Wear Scar X"() -> (w3797:dbl)
                "Length ( microns ) 2" <- w3797
                n3013 = local read "Wear Scar Y"() -> (w3796:dbl)
                "Wear Scar Y ( microns ) :" <- w3796
                n3014 = local read "Test Date 2"() -> (w3826:string)
                n3015 = local read "Tested by 2"() -> (w3827:string)
                n3016 = local read "String 46"() -> (w3823:string)
                n3017 = local read "String 48"() -> (w3829:string)
                n3018 = local read "String 47"() -> (w3828:string)
                n3019 = local read "String 49"() -> (w3830:string)
                n3020 = local read "String 10"() -> (w3783:string)
                n3021 = local read "s.NO 2"() -> (w3824:string)
                n3022 = Add(x=w3797, y=w3796) -> (x+y=w3795:dbl)
                n3023 = call <vilib>:"New Report.vi"("report type"=enum16{"Standard Report", "HTML"}."HTML") -> ("report out"=w3803:refnum<class "NI_report.lvclass">, "error out"=w3801:errorcluster)  [unwired: 13 in]
                n3024 = Concatenate Strings(w3832, w3823, w3824, w3832, w3829, w3825, w3832, w3828, w3826, w3832, w3830, w3827, w3832) -> (→"test by 2":string)
                n3025 = Concatenate Strings("C:\\LAB-IQ\\Data\\" ("string"), w3783, ".jpg" ("string")) -> ()  [unwired: 1 out]
                n3026 = Divide(x=w3795, y=2.0) -> (x/y=→"Mean Wear ( microns) :":dbl)
                n3027 = call-dynamic "Set Report Orientation.vi"("report in"=w3803, "orientation (portrait)"=w3799, "error in (no error)"=w3801) -> ("report out"=w3802:refnum<class "NI_report.lvclass">, "error out"=w3800:errorcluster)  [unwired: 11 in]
                n3028 = for {
                  N: 5 -> [_]
                  tunnel: w3802 -> [w3853]
                  tunnel: [w3852] -> w3781
                  tunnel: w3800 -> [w3851]
                  tunnel: [w3850] -> w3780
                  n3029 = call-dynamic "Set Report Tab Width.vi"("report in"=w3853, "error in (no error)"=w3851) -> ("report out"=w3852:refnum<class "NI_report.lvclass">, "error out"=w3850:errorcluster)  [unwired: 12 in]
                }
                n3030 = local read "TITTLE"() -> (w3798:string)
                n3031 = call-dynamic "Set Report Header Text.vi"("report in"=w3781, "center header text"=w3798, "error in (no error)"=w3780) -> ("report out"=w3819:refnum<class "NI_report.lvclass">, "error out"=w3818:errorcluster)  [unwired: 11 in]
                n3032 = for {
                  N: 1 -> [_]
                  tunnel: [w3857] -> w3805
                  tunnel: [w3856] -> w3804
                  tunnel: w3819 -> [w3855]
                  tunnel: w3818 -> [w3854]
                  n3033 = call-dynamic "New Report Line.vi"("report in"=w3855, "error in (no error)"=w3854) -> ("report out"=w3857:refnum<class "NI_report.lvclass">, "error out"=w3856:errorcluster)  [unwired: 12 in]
                }
                n3034 = for {
                  N: 2 -> [_]
                  tunnel: [w3849] -> w3811
                  tunnel: [w3848] -> w3810
                  tunnel: w3805 -> [w3847]
                  tunnel: w3804 -> [w3846]
                  n3035 = call-dynamic "New Report Line.vi"("report in"=w3847, "error in (no error)"=w3846) -> ("report out"=w3849:refnum<class "NI_report.lvclass">, "error out"=w3848:errorcluster)  [unwired: 12 in]
                }
                n3036 = for {
                  N: 25 -> [_]
                  tunnel: w3811 -> [w3845]
                  tunnel: w3810 -> [w3843]
                  tunnel: [w3844] -> w3814
                  tunnel: [w3842] -> w3813
                  n3037 = call-dynamic "Set Report Tab Width.vi"("report in"=w3845, "error in (no error)"=w3843) -> ("report out"=w3844:refnum<class "NI_report.lvclass">, "error out"=w3842:errorcluster)  [unwired: 12 in]
                }
                n3038 = control-ref of="Tab Control 9"() -> (w3809:refnum<vi>)
                n3039 = call-dynamic "Append Control Image to Report.vi"("report in"=w3814, "alignment (default)"=HTML_Report_Image_Alignment."ABSMIDDLE", "ctrl reference"=w3809, "error in (no error)"=w3813) -> ("report out"=w3808:refnum<class "NI_report.lvclass">, "error out"=w3807:errorcluster)  [unwired: 8 in, 2 out]
                n3040 = for {
                  N: 3 -> [_]
                  tunnel: [w3841] -> w3792
                  tunnel: [w3840] -> w3791
                  tunnel: w3808 -> [w3839]
                  tunnel: w3807 -> [w3838]
                  n3041 = call-dynamic "New Report Line.vi"("report in"=w3839, "error in (no error)"=w3838) -> ("report out"=w3841:refnum<class "NI_report.lvclass">, "error out"=w3840:errorcluster)  [unwired: 12 in]
                }
                n3042 = for {
                  N: 100 -> [_]
                  tunnel: w3792 -> [w3837]
                  tunnel: w3791 -> [w3835]
                  tunnel: [w3836] -> w3788
                  tunnel: [w3834] -> w3786
                  n3043 = call-dynamic "Set Report Tab Width.vi"("report in"=w3837, "error in (no error)"=w3835) -> ("report out"=w3836:refnum<class "NI_report.lvclass">, "error out"=w3834:errorcluster)  [unwired: 12 in]
                }
                n3044 = String To Path(string="C:\\LAB-IQ\\im\\Temp_resized.jpg") -> (path=w3778:path)
                n3045 = call-poly <vilib>:"Append Image to Report.vi"("report in"=w3788, "path or URL of image"=w3778, "error in (no error)"=w3786) -> ("report out"=w3787:refnum<class "NI_report.lvclass">, "error out"=w3785:errorcluster)  [unwired: 9 in, 2 out]
                n3046 = call-poly <vilib>:"Open HTML Report in Browser.vi"("report in"=w3787, "error in (no error)"=w3785) -> ("report out"=w3822:refnum<class "NI_report.lvclass">, "error out"=w3821:errorcluster)  [unwired: 11 in, 1 out]
                n3047 = call-dynamic "Dispose Report.vi"("report in"=w3822, "error in (no error)"=w3821) -> ()  [unwired: 13 in, 1 out]
              }
              frame #2 {
              }
              frame #3 {
                n3048 = disable-structure shown="Disabled" {
                  frame Disabled {
                    n3049 = local read "String 10"() -> (w3862:string)
                    n3050 = Concatenate Strings("C:\\LAB-IQ-NXT\\Data\\" ("string"), w3862, ".jpg" ("string")) -> (w3860:string)
                    n3051 = String To Path(string=w3860) -> (path=w3859:path)
                    n3052 = Delete(path (use dialog)=w3859) -> ()  [unwired: 4 in, 3 out]
                  }
                  frame Enabled {
                  }
                }
                n3053 = local write "Print 2"(FALSE ("Print")) -> ()
              }
            }
          }
        }
      }
    }
    n3054 = Wait (ms)(milliseconds to wait=u32 50) -> ()  [unwired: 1 out]
    n3055 = Wait (ms)(milliseconds to wait=u32 50) -> ()  [unwired: 1 out]
    n3056 = local read "Quit"() -> (w2196:bool)
  }
  n3057 = VISA Close(VISA resource name=w41, error in (no error)=w40) -> ()  [unwired: 1 out]
  n3058 = while {
    stop <- w4013 stop-if-true
    n3059 = local read "Auto Start Test"() -> (w4011:bool)
    n3060 = local read "RUN"() -> (w4010:bool)
    n3061 = Wait (ms)(milliseconds to wait=u32 1000) -> ()  [unwired: 1 out]
    n3062 = Or(x=w4010, y=w4011) -> (x .or. y?=w4009:bool)
    n3063 = case shown="True" w4009 {
      frame False {
      }
      frame True {
        n3064 = local read "LVDT STROKE Actual"() -> (w4014:dbl)
        n3065 = In Range and Coerce(upper limit=1.2, x=w4014, lower limit=0.6) -> (In Range?=w4017:bool)  [unwired: 1 out]
        n3066 = call-poly <vilib>:"Random Number (Range).vi"("lower bound (0)"=0.998 ("upper bound (100)"), "upper bound (100)"=1.003) -> ("number"=w4015:dbl)  [unwired: 9 in]
        n3067 = case shown="True" w4017 {
          tunnel: [w4022 w4023] -> w4016
          tunnel: w4015 -> [_ w4023]
          tunnel: w4014 -> [w4022 _]
          frame False {
          }
          frame True {
          }
        }
        "LVDT STROKE DISPLAY" <- w4016
      }
    }
    n3068 = local read "Quit"() -> (w4013:bool)
  }
  n3069 = while {
    tunnel: [w4040] -> w49
    shift-right: [w4033] -> _
    shift-left: 0.0 -> [w4036]
    shift-right: [w4032] -> _
    shift-left: 0.0 -> [w4035]
    shift-right: [w4031] -> _
    shift-left: 100.0 ("vc_cmd") -> [w4034]
    stop <- w4040 stop-if-true
    # "PID LOGIC"
    n3070 = local read "run test Calibration"() -> (w4028:bool)
    n3071 = local read "RUN"() -> (w4038:bool)
    n3072 = local read "Auto Start Temp"() -> (w4029:bool)
    n3073 = local read "Auto Start Test"() -> (w4037:bool)
    n3074 = local read "START TEMP"() -> (w4027:bool)
    n3075 = And(x=w4029, y=w4037) -> (x .and. y?=w4030:bool)
    n3076 = Or(x=w4038, y=w4030) -> (x .or. y?=w4039:bool)
    n3077 = And(x=w4039, y=w4027) -> (x .and. y?=w4026:bool)
    n3078 = And(x=w4028, y=w4027) -> (x .and. y?=w4025:bool)
    n3079 = Or(x=w4025, y=w4026) -> (x .or. y?=w4024:bool)
    n3080 = Wait (ms)(milliseconds to wait="milliseconds to wait") -> ()  [unwired: 1 out]
    n3081 = case shown="True" w4024 {
      tunnel: [400.0 ("out_vc_cmd") w4059] -> w4031
      tunnel: [w4043 w4061] -> w4032
      tunnel: [w4043 w4060] -> w4033
      tunnel: w4036 -> [_ w4050]
      tunnel: w4035 -> [_ w4049]
      tunnel: w4034 -> [_ w4048]
      tunnel: w4028 -> [_ w4044]
      frame False {
        w4043 = 0.0 ("error_out")
      }
      frame True {
        n3082 = case shown="True" w4044 {
          tunnel: [w4068 1.0] -> w4046
          frame False {
            n3083 = local read "Set Strk"() -> (w4067:dbl)
            n3084 = Add(x=w4067, y="Add up Stroke") -> (x+y=w4068:dbl)
          }
          frame True {
          }
        }
        n3085 = local read "LVDT STROKE"() -> (w4045:dbl)
        n3086 = formula code="// Zero-Hardcode Explicit Positional-Form PID Engine\n// Inputs: target_stroke, measured_stroke, dt, prev_error, integral_accumulator_in, prev_vc_cmd\n//         kp, ki, kd, max_step_change, max_amplitude, min_amplitude, startup_cmd\n// Outputs: vc_cmd, error_out, out_error, integral_accumulator_out, out_vc_cmd\n\n// 1. Calculate Tracking Error\nfloat current_error = target_stroke - measured_stroke;\nerror_out = current_error;\n\n// 2. Compute Proportional Term\nfloat p_term = kp * current_error;\n\n// 3. Compute Derivative Term\nfloat d_term = 0.0;\nif (dt > 0.0) {\n    d_term = kd * ((current_error - prev_error) / dt);\n}\n\n// 4. Update and Accumulate Integral Term\nfloat current_integral = integral_accumulator_in + (current_error * dt);\nfloat i_term = ki * current_integral;\n\n// 5. Calculate Ideal Target Command (Anchored by startup baseline)\nfloat ideal_command = startup_cmd + p_term + i_term + d_term;\n\n// 6. Apply Loop Rate Limiting FIRST \n// (Forces the command to climb gradually from prev_vc_cmd instead of jumping straight to max)\nfloat raw_adjustment = ideal_command - prev_vc_cmd;\n\nif (raw_adjustment > max_step_change) {\n    raw_adjustment = max_step_change;\n} else if (raw_adjustment < -max_step_change) {\n    raw_adjustment = -max_step_change;\n}\n\nfloat next_vc_cmd = prev_vc_cmd + raw_adjustment;\n\n// 7. Anti-Windup Protection & Final Output Safety Safeguard Clamping\n// (Back-calculating based on what we are ACTUALLY outputting)\nif (next_vc_cmd > max_amplitude) {\n    float excess = next_vc_cmd - max_amplitude;\n    if (ki > 0.0) {\n        current_integral -= excess / ki;\n    }\n    next_vc_cmd = max_amplitude;\n} else if (next_vc_cmd < min_amplitude) {\n    float excess = next_vc_cmd - min_amplitude;\n    if (ki > 0.0) {\n        current_integral -= excess / ki;\n    }\n    next_vc_cmd = min_amplitude;\n}\n\n// 8. Map to Shift Registers for memory persistence\nvc_cmd = next_vc_cmd;\nout_error = current_error;                   \nintegral_accumulator_out = current_integral;  \nout_vc_cmd = next_vc_cmd;"("target_stroke"=w4046, "measured_stroke"=w4045, "dt"="dt", "integral_accumulator_in"=w4049, "prev_error"=w4050, "prev_vc_cmd"=w4048, "kp"="kp", "ki"="ki", "kd"="kd", "max_step_change"="max_step_change", "max_amplitude"="max_amplitude", "min_amplitude"="min_amplitude", "startup_cmd"="startup_cmd") -> ("vc_cmd"=w4065:dbl, "out_error"=w4060:dbl, "integral_accumulator_out"=w4061:dbl, "out_vc_cmd"=w4059:dbl)  [unwired: 1 out]